vi "Minhee Analysis.vi"(5 "Data type":T4 items=["AXON", "HEKA", "TEXT"], 7 "Path of File":path=path "C:/Users/KimYG/Desktop/test4.abf") -> ()   [LabVIEW 2017] (continued)
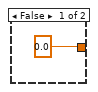
[diagram p4: hidden frame]
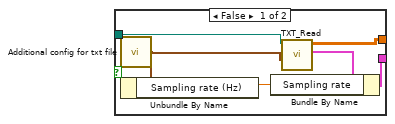
[diagram p5: hidden frame]
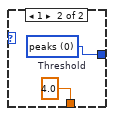
[diagram p6: hidden frame]
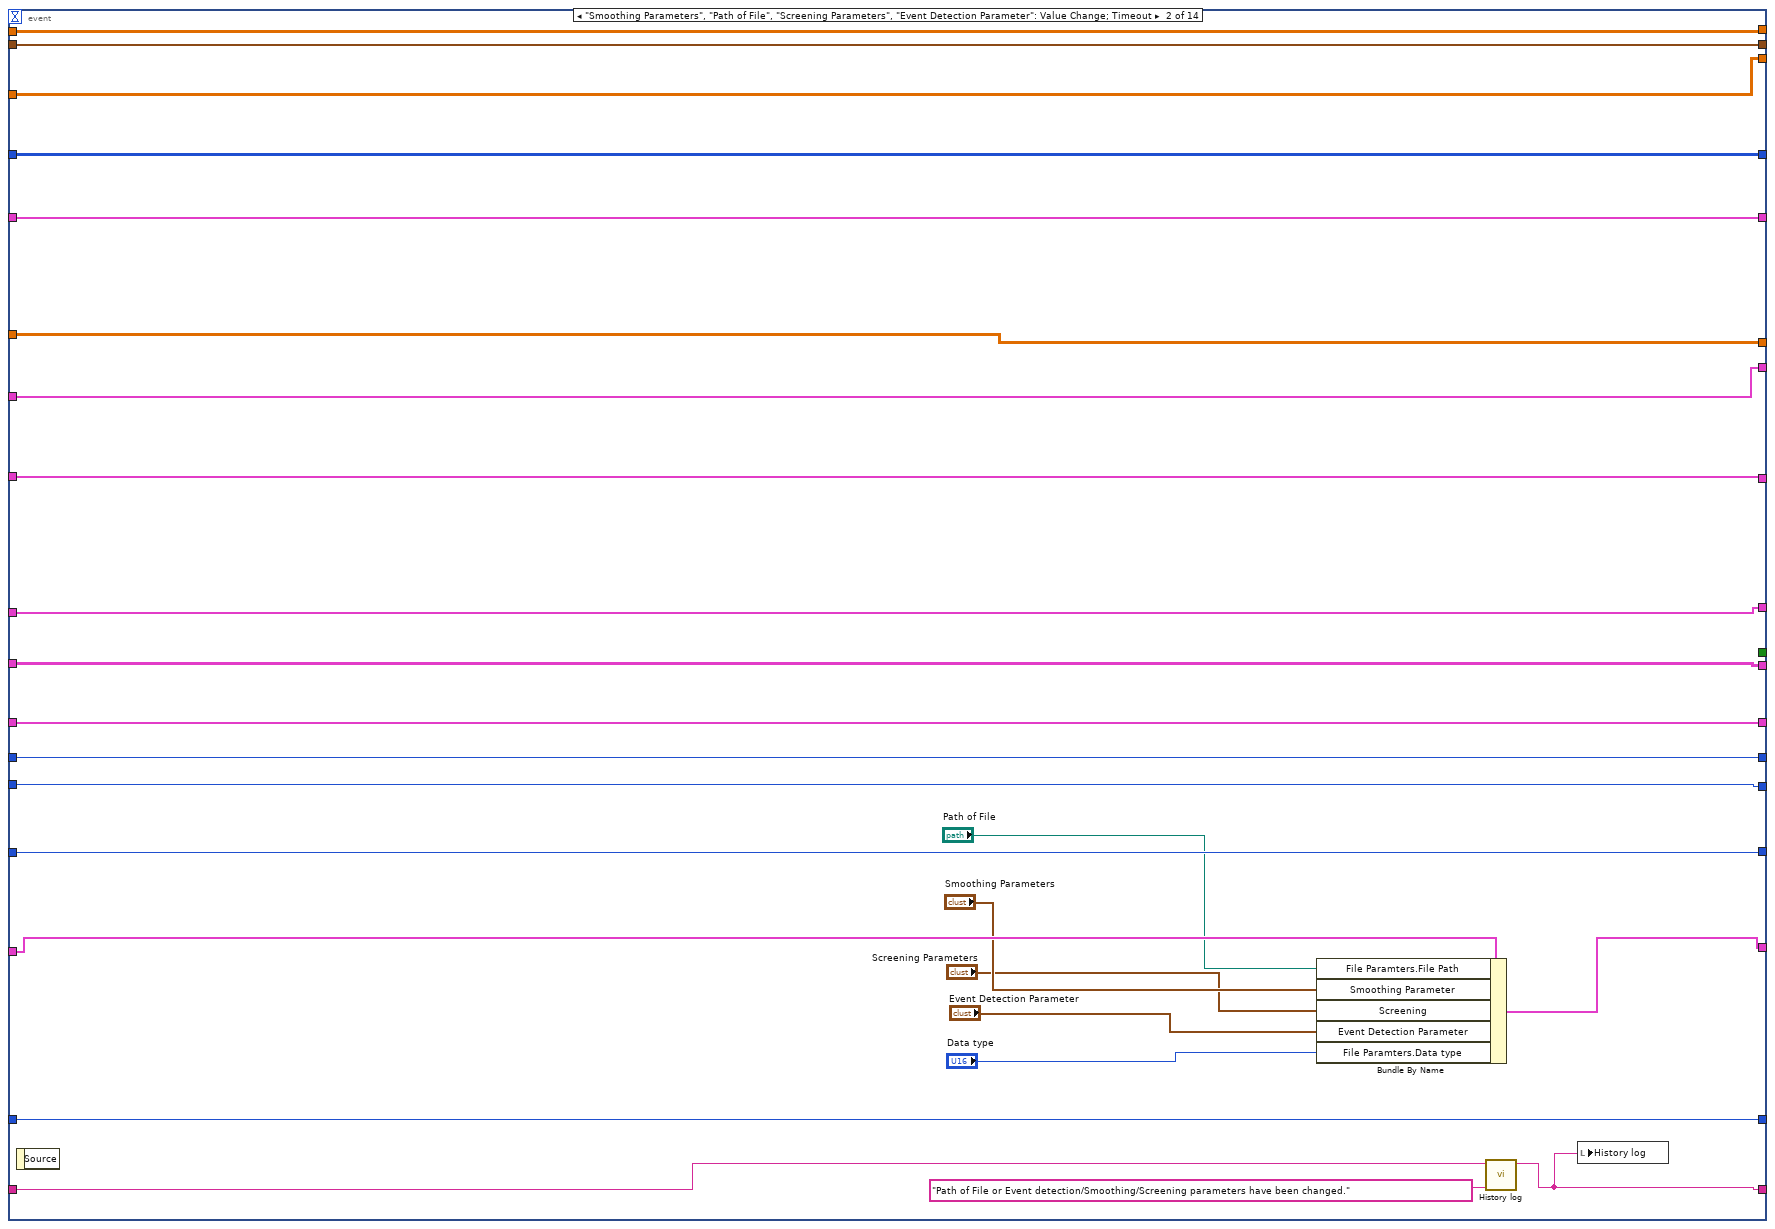
[diagram p7: hidden frame]
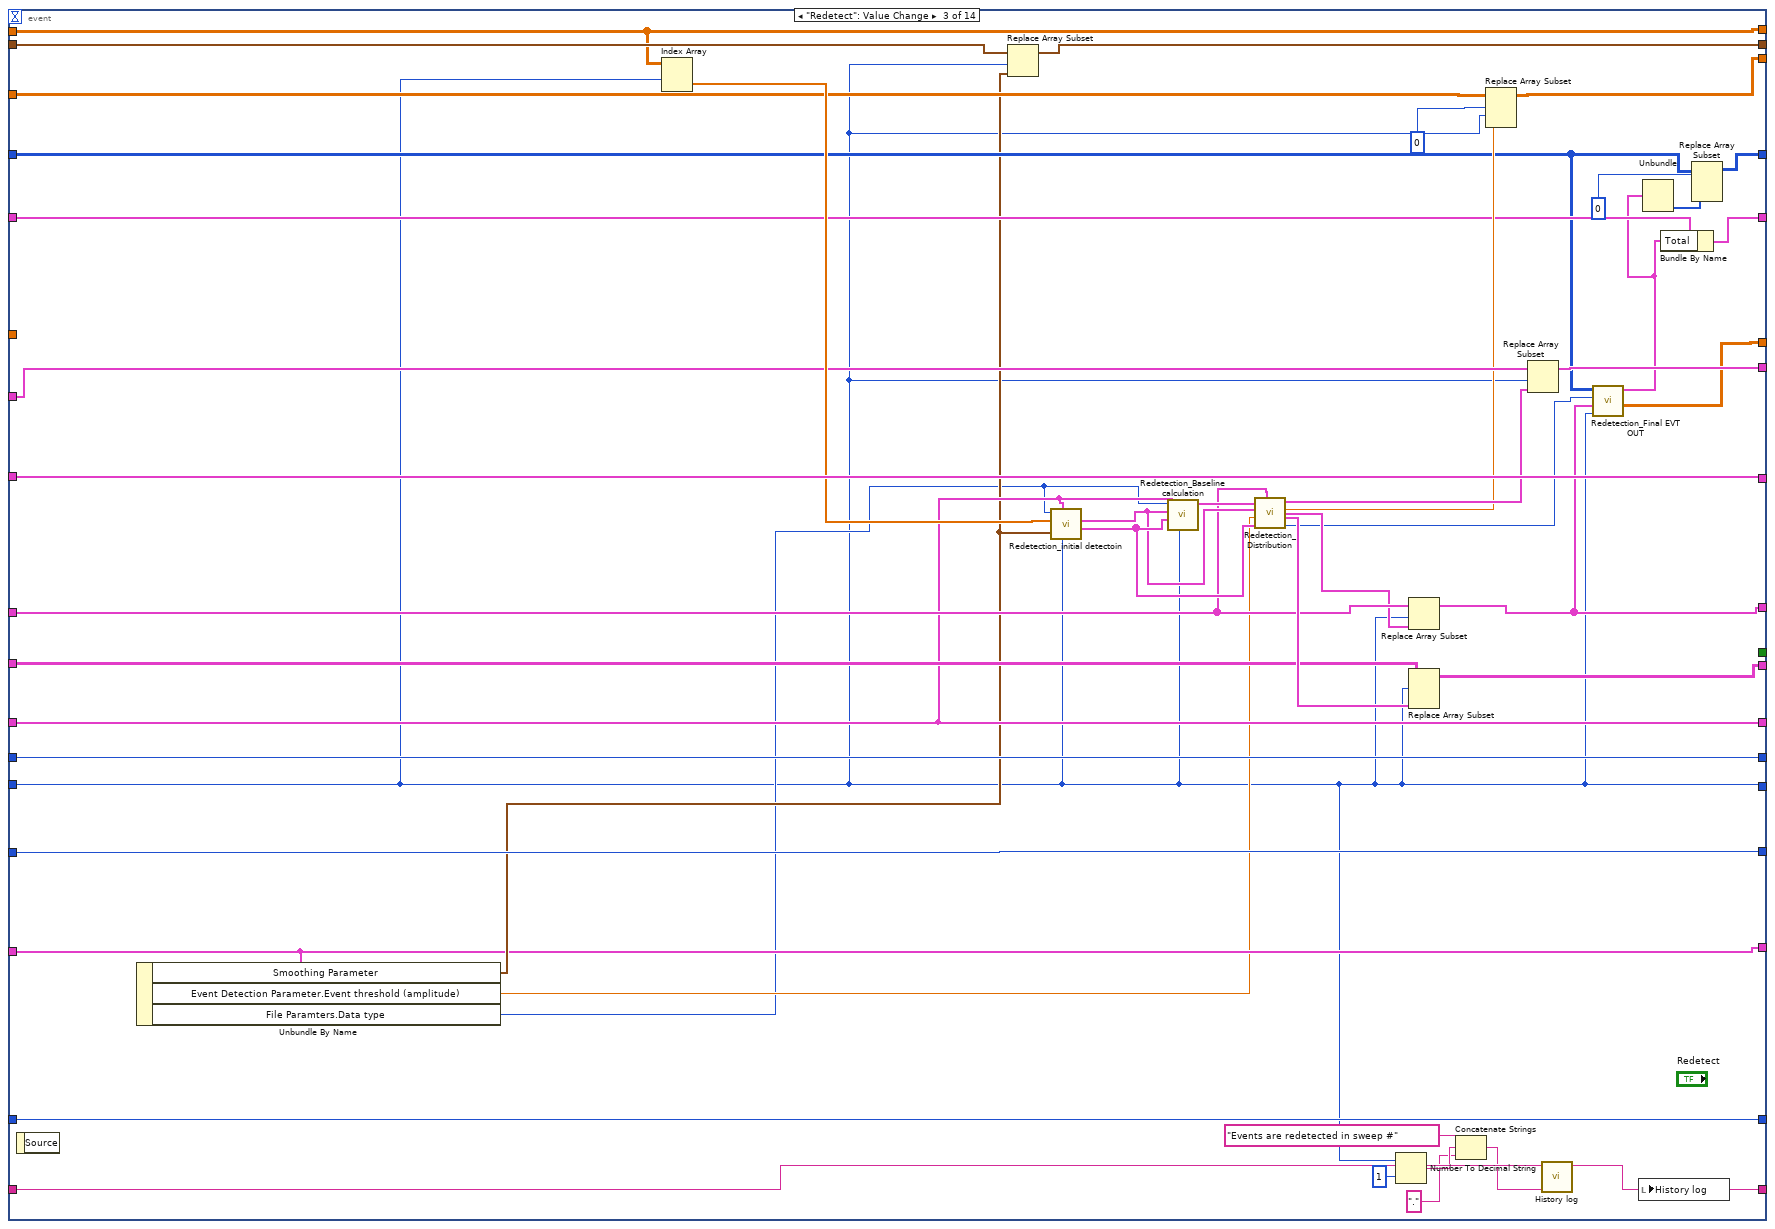
[diagram p8: hidden frame]
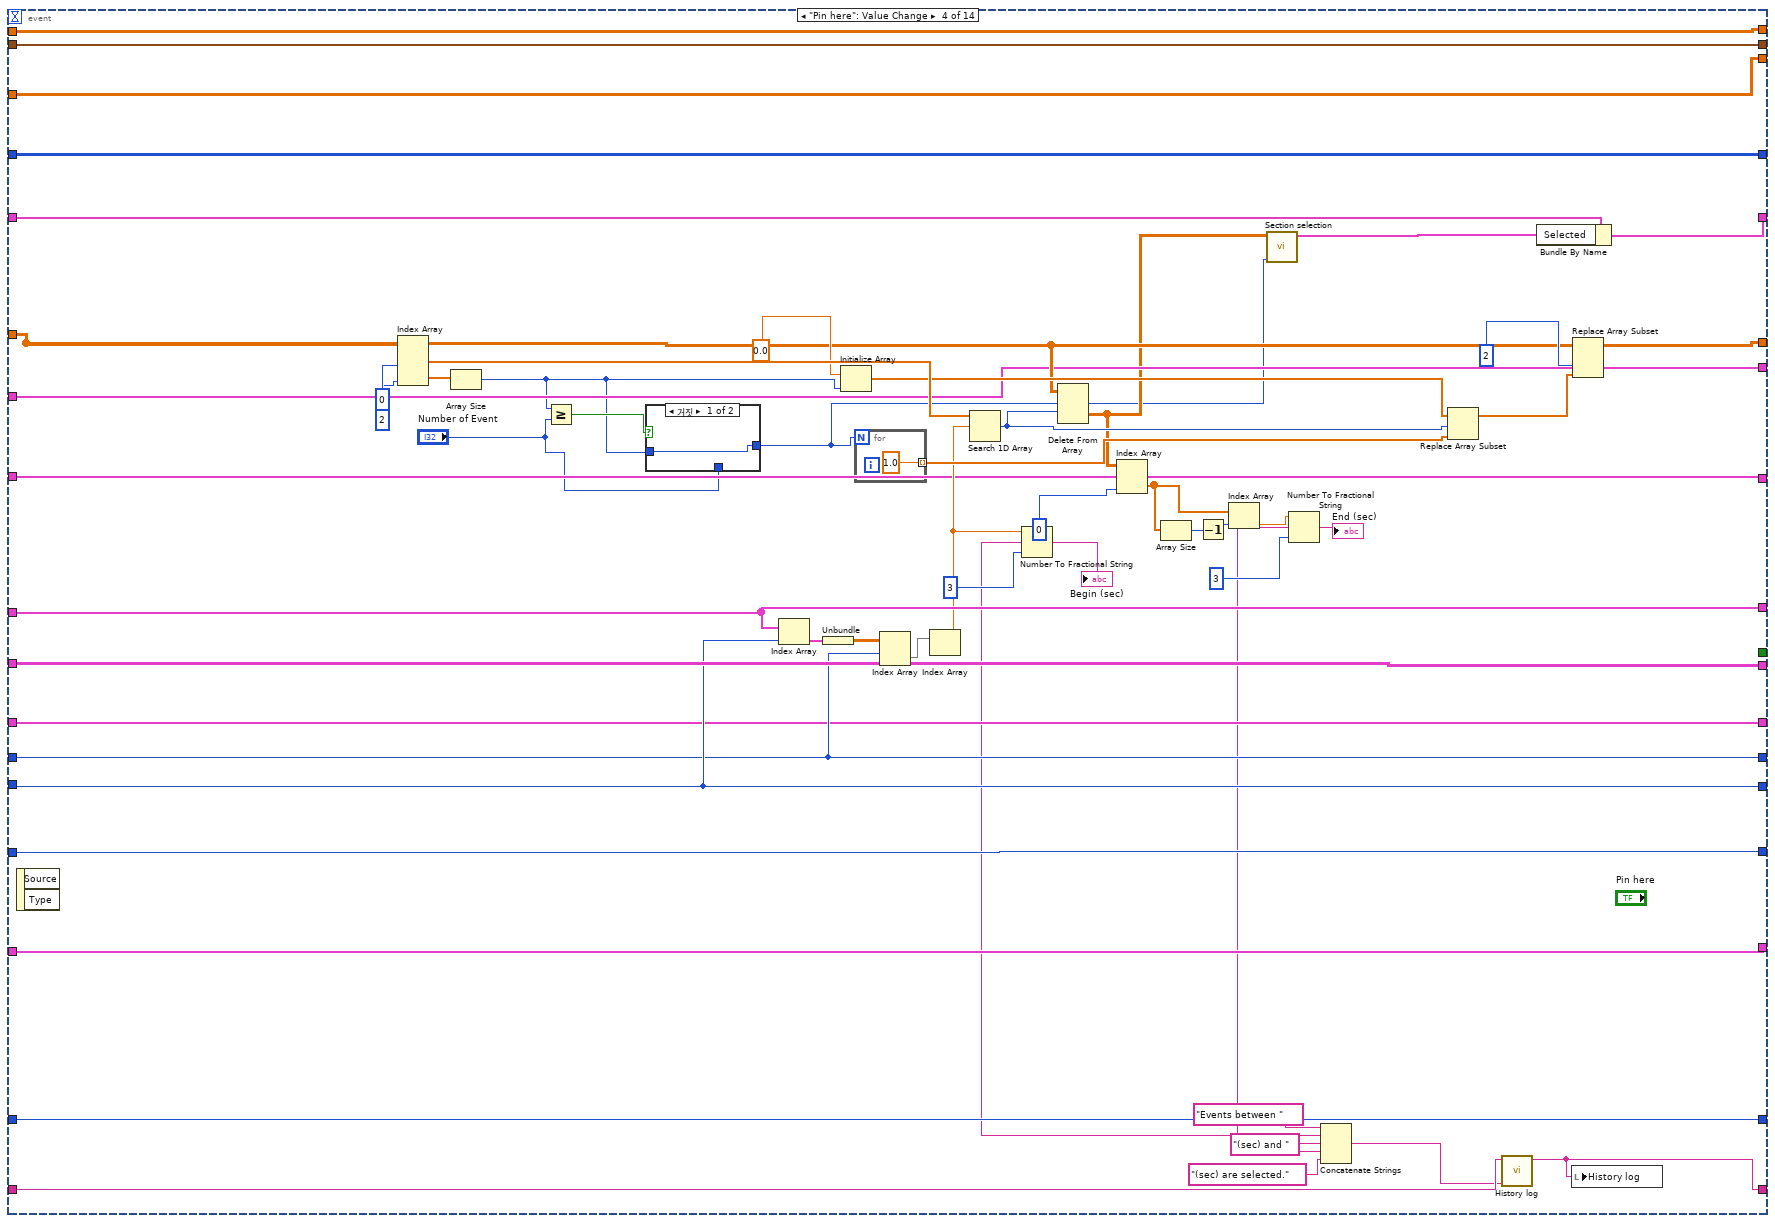
[diagram p9: hidden frame]
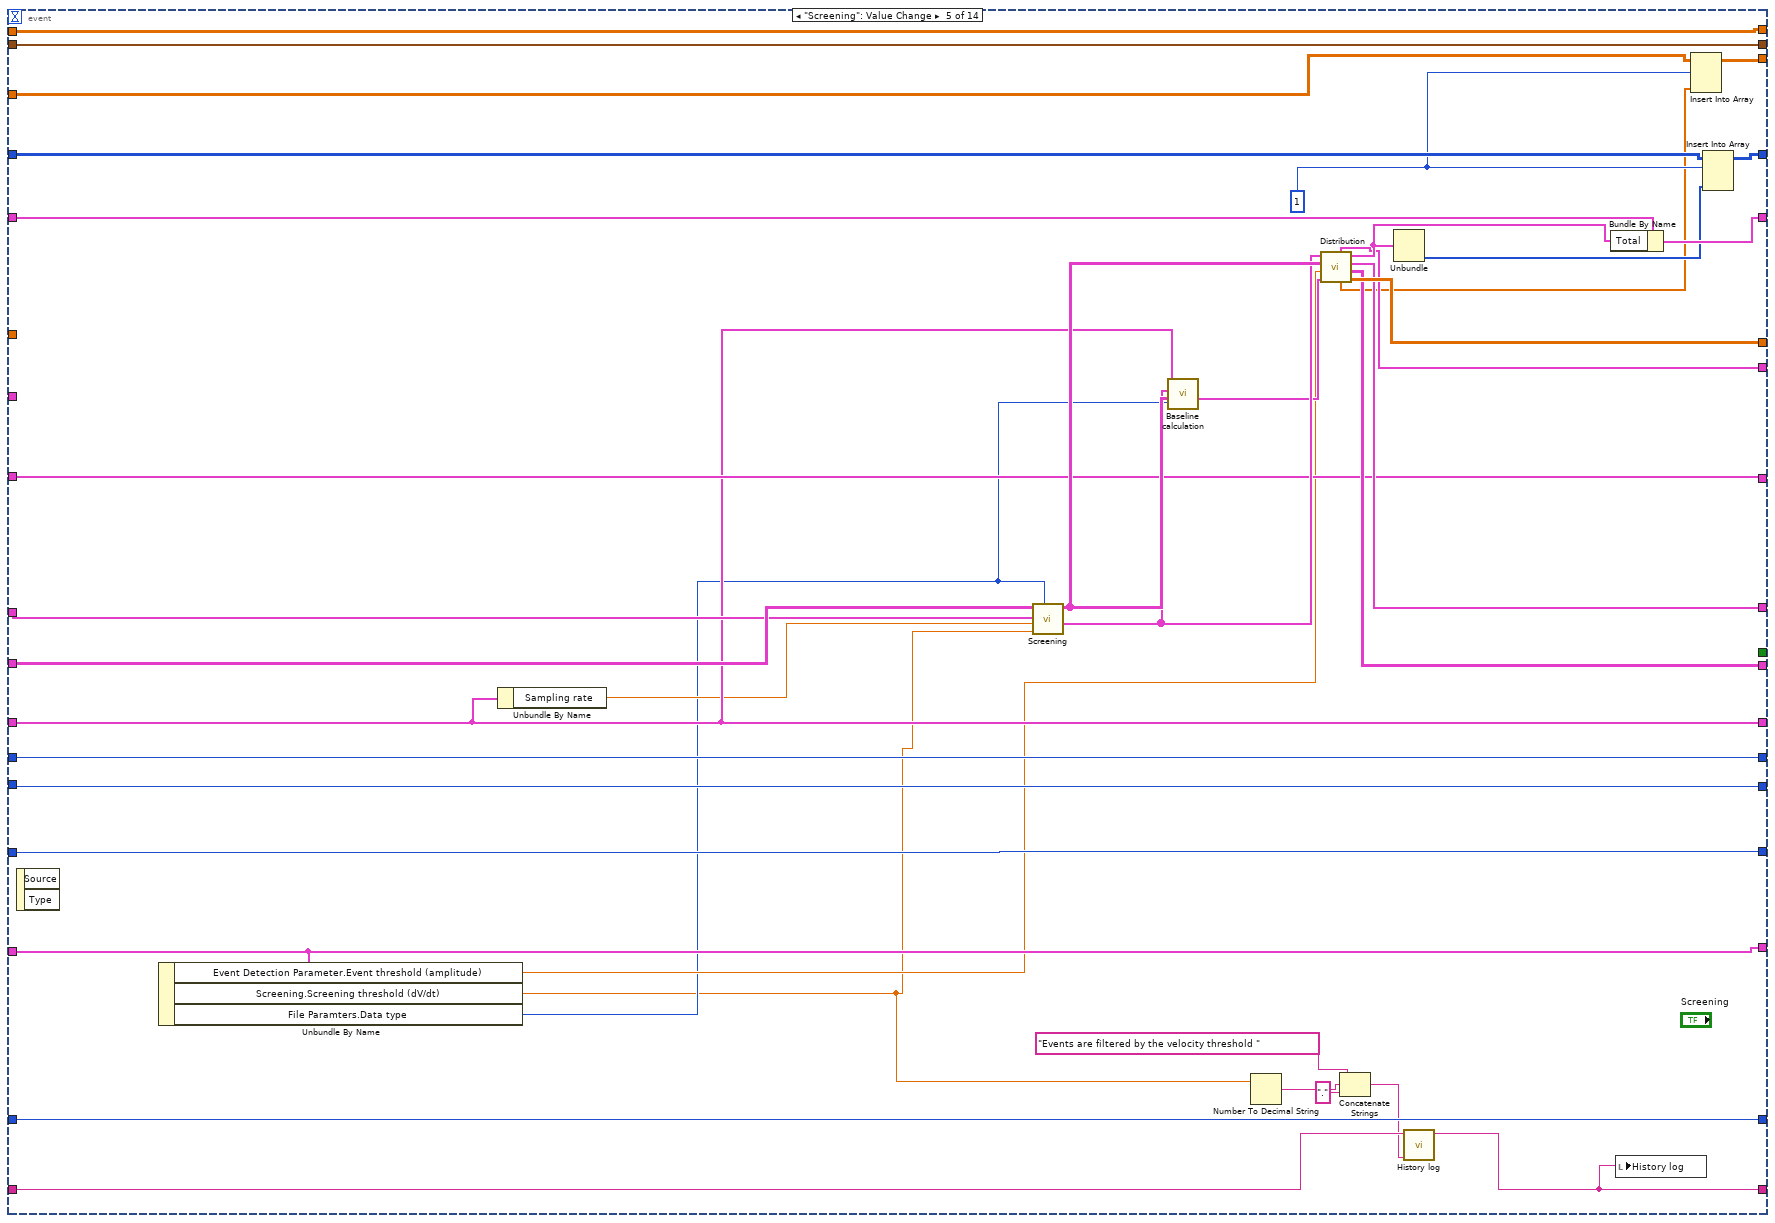
[diagram p11: hidden frame]
            n155 = Number To Decimal String(number=w476) -> (decimal integer string=w474:string)  [unwired: 1 in]
            n156 = call "Distribution.vi"("Detected Event IN"=w497, "Sweep trace (2D) In"=w491, "Threshold"=w479, "Baseline info IN"=w492) -> ("Baseline info new OUT"=w488:cluster{dbl[][]}[], "Distribution (output)"=w495:T15, "Detected Event (1D) OUT"=w489:cluster{dbl[][]}[], "Sweep trace (2D) Out"=w490:cluster{"Ramp Pattern":dbl[], "X":dbl[]}[][], "Event final OUT"=w496:dbl[][])  [unwired: 1 out]
            n157 = Concatenate Strings("Event is deleted. ", " (Event #", w474, " in Sweep #", w471, ")" ("문자열")) -> (w469:string)
            n158 = call "History log.vi"("Message"=w469, "String IN"=w477) -> ("String OUT"=w468:string)  [unwired: 5 in]
            n159 = local write "History log"(w468) -> ()
            n160 = Bundle By Name(cluster=w494, "Total"=w495) -> (w493:T7)
          }
          event "Clipboard": Value Change {
            n161 = event-data() -> ()  [unwired: 1 in, 2 out]
            n162 = Unbundle By Name(w505) -> ("File Paramters.Data type"=w504:T4)
            n163 = case shown="1" w504 {
              tunnel: w513 -> [w526 w533]
              tunnel: [w526 w532] -> w514
              frame 0, Default {
              }
              frame 1 {
                n164 = Index Array(array=w533, index (col)=0 ("비활성화된 인덱스 (열)")) -> (element=w530:dbl[])  [unwired: 1 in]
                n165 = Divide(x=w530, y=2.0 ("x")) -> (x/y=w528:dbl[])
                n166 = Replace Array Subset(array=w533, new element=w528, index (col)=0 ("비활성화된 인덱스 (열)")) -> (w532:dbl[][])  [unwired: 1 in]
              }
            }
            n167 = Number To Exponential String(number=w514) -> (E-format string=w516:string[][])  [unwired: 3 in]
            n168 = call <userlib>:"Clipboard transformation.vi"("Input (structured)"=w516) -> ("Output (flattened)"=w517:string)  [unwired: 1 in, 1 out]
            n169 = Open Application Reference() -> (0:w519:errorcluster)  [unwired: 4 in, 1 out]
            n170 = invoke class="App" method="Clipboard.Write"(error in=w519, "Param 0"=w517) -> (reference out=w518:refnum<vi>)  [unwired: 2 in, 3 out]
            n171 = call "History log.vi"("Message"="Events are exported to clipboard.", "String IN"=w503) -> ("String OUT"=w501:string)  [unwired: 5 in]
            n172 = Close Reference(reference=w518) -> ()  [unwired: 1 in, 1 out]
            n173 = local write "History log"(w501) -> ()
          }
          event "Event #": Value Change {
            n174 = event-data() -> ()  [unwired: 1 in, 1 out]
          }
          event "Trace to display", "Derivative": Value Change {
            n175 = event-data() -> ()  [unwired: 1 in, 1 out]
          }
          event "File Explorer": Value Change {
            n176 = event-data() -> ()  [unwired: 1 in, 1 out]
            n177 = Unbundle By Name(w570) -> ("File Paramters.File Path"=w569:path)
            n178 = call <vilib>:"Show in File System.vi"("file or directory path"=w569) -> ()  [unwired: 10 in, 1 out]
          }
          event "Raw trace": Value Change {
            w605 = TRUE ("눈금 숨기기")
            n179 = event-data() -> ()  [unwired: 1 in, 2 out]
            n180 = Index Array(array=w614, index (row)=w613) -> (element=w612:cluster{"Ramp Pattern":dbl[], "X":dbl[]}[])  [unwired: 1 in]
            n181 = Index Array(array=w612, index=1 ("인덱스")) -> (element=w610:cluster{"Ramp Pattern":dbl[], "X":dbl[]})
            n182 = Unbundle(w610) -> ("Ramp Pattern"=w609:dbl[], "X"=w608:dbl[])
            n183 = Build Array(w609, w608) -> (w607:dbl[][])
            n184 = call-poly <vilib>:"Write Delimited Spreadsheet.vi"("2D data"=w607, "transpose? (no:F)"=TRUE ("transpose? (F)")) -> ("new file path (Not A Path if cancelled)"=w602:path, "error out"=w598:errorcluster)  [unwired: 12 in]
            n185 = Strip Path(path=w602) -> (stripped path=w601:path)  [unwired: 1 out]
            n186 = Build Path(base path=w601, name or relative path="Raw trace.bmp" ("이름 또는 상대 경로")) -> (appended path=w599:path)
            n187 = invoke on="Whole trace" class="XYGraph (엄격한)" method="Export Image"(error in=w598, "FileType"=enum32{"BMP", "EPS", "EMF", "PICT"}."BMP" ("파일 타입"), "Target"=enum32{"File", "Clipboard"}."File" ("타겟"), "Path"=w599, "HideGrid"=w605, "Overwrite"=w605) -> ()  [unwired: 2 in, 8 out]
          }
          event "Save": Value Change {
            n188 = event-data() -> ()  [unwired: 1 in, 2 out]
            n189 = Unbundle By Name(w627) -> ("File Paramters.File Path"=w626:path, "File Paramters.Data type"=w625:T4)
            n190 = Strip Path(path=w626) -> (stripped path=w644:path, name=w640:string)
            n191 = case shown="0, 기본" w625 {
              tunnel: w642 -> [w654 w661]
              tunnel: [w654 w660] -> w641
              frame 0, Default {
              }
              frame 1 {
                n192 = Index Array(array=w661, index (col)=0 ("비활성화된 인덱스 (열)")) -> (element=w658:dbl[])  [unwired: 1 in]
                n193 = Divide(x=w658, y=2.0 ("x")) -> (x/y=w656:dbl[])
                n194 = Replace Array Subset(array=w661, new element=w656, index (col)=0 ("비활성화된 인덱스 (열)")) -> (w660:dbl[][])  [unwired: 1 in]
              }
            }
            n195 = To Lower Case(string=w640) -> (all lower case string=w639:string)
            n196 = Match Pattern(string=w639, regular expression="abf" ("정규식")) -> (before substring=w647:string)  [unwired: 1 in, 3 out]
            n197 = Concatenate Strings(w647, "txt" ("문자열")) -> (w645:string)
            n198 = Build Path(base path=w644, name or relative path=w645) -> (appended path=w643:path)
            n199 = call-poly <vilib>:"Write Delimited Spreadsheet.vi"("file path (dialog if empty)"=w643, "format (%.3f)"="%.5f", "2D data"=w641, "transpose? (no:F)"=FALSE ("transpose? (F)")) -> ("new file path (Not A Path if cancelled)"=w623:path)  [unwired: 10 in, 1 out]
            n200 = Path To String(path=w623) -> (string=w621:string)
            n201 = Concatenate Strings("Event file is saved. (file path: ", w621, ")") -> (w619:string)
            n202 = call "History log.vi"("Message"=w619, "String IN"=w624) -> ("String OUT"=w618:string)  [unwired: 5 in]
            n203 = local write "History log"(w618) -> ()
          }
          event Panel Close? {
            n204 = event-data() -> ()  [unwired: 1 in, 4 out]
            n205 = Two Button Dialog(message="Are you sure you want to quit?" ("메시지"), 1:"Cancel" ("거짓 버튼 이름(\"취소\")"), 2:"Yes" ("참 버튼 이름(\"확인\")")) -> (T button?=w683:bool)
            n206 = case shown="참" w683 {
              tunnel: [FALSE TRUE] -> w701
              tunnel: w699 -> [w720 _]
              tunnel: w698 -> [w719 _]
              tunnel: w697 -> [w718 _]
              tunnel: w696 -> [w717 _]
              tunnel: w695 -> [w715 _]
              tunnel: w694 -> [w714 w729]
              tunnel: w693 -> [w713 w728]
              tunnel: [w720 _] -> w692
              tunnel: [w719 _] -> w691
              tunnel: [w718 _] -> w690
              tunnel: [w717 _] -> w689
              tunnel: w688 -> [w716 w724]
              tunnel: [w716 w724] -> w687
              tunnel: [w715 _] -> w686
              tunnel: [w714 w729] -> w685
              tunnel: [w713 w728] -> w684
              tunnel: w682 -> [w711 _]
              tunnel: [w711 _] -> w681
              tunnel: w680 -> [w710 _]
              tunnel: [w710 _] -> w679
              tunnel: w678 -> [w709 _]
              tunnel: [w709 _] -> w677
              tunnel: w676 -> [w708 _]
              tunnel: [w708 u16 0 ("Trace to display")] -> w675
              tunnel: w674 -> [w707 _]
              tunnel: [w707 _] -> w673
              tunnel: w672 -> [w706 _]
              tunnel: [w706 _] -> w671
              tunnel: w670 -> [w705 _]
              tunnel: [w705 _] -> w669
              tunnel: w666 -> [w704 _]
              tunnel: [w704 _] -> w665
              tunnel: w664 -> [w703 w722]
              tunnel: [w703 w722] -> w663
              tunnel: [TRUE TRUE] -> w662
              frame False {
              }
              frame True {
                w725 = ""
                w726 = dbl[] [] ("CV")
                n207 = property on="Begin (sec)" class="Str"("Value"=w725) -> ()  [unwired: 2 in, 2 out]
                n208 = property on="End (sec)" class="Str"("Value"=w725) -> ()  [unwired: 2 in, 2 out]
                n209 = property on="CV" class="WFGraph (엄격한)"("Value"=w726) -> ()  [unwired: 2 in, 2 out]
                n210 = property on="Holding Current" class="WFGraph (엄격한)"("Value"=w726) -> ()  [unwired: 2 in, 2 out]
              }
            }
            n211 = event-data("Discard?"=w662) -> ()  [unwired: 1 in, 1 out]
          }
        }
        "Number of event" <- w89
        "Averaged Amplitude" <- w62
        n212 = Unbundle By Name(w103) -> ("Total.Distribution of IEI"=→"Distribution of IEI":T5, "Total.Distribution of amplitude"=→"Distribution of amplitude":T5, "Total.Total"=w100:T19, "Selected.Distribution of IEI"=→"Distribution of IEI 2":T5, "Selected.Distribution of amplitude"=→"Distribution of amplitude 2":T5, "Selected.Selected"=w94:T20)
        n213 = Unbundle By Name(w34) -> ("Screening.Screening threshold (dV/dt)"=w33:dbl, "File Paramters.Data type"=w32:T4)
        n214 = Unbundle By Name(w87) -> ("Sampling rate"=w86:dbl)
        n215 = Index Array(array=w137, index (row)=w37) -> (element=w73:cluster{"Ramp Pattern":dbl[], "X":dbl[]}[])  [unwired: 1 in]
        n216 = Index Array(array=w73, index=2 ("인덱스")) -> (element=w112:cluster{"Ramp Pattern":dbl[], "X":dbl[]})
        n217 = local read "Sweep duration"() -> (w84:dbl)
        n218 = Unbundle By Name(w112) -> ("X"=w66:dbl[])
        n219 = Index Array(array=w73, index #1=0 ("인덱스"), index #2=2 ("인덱스"), index #3=1 ("인덱스")) -> (element #1=w70:cluster{"Ramp Pattern":dbl[], "X":dbl[]}, element #2=w68:cluster{"Ramp Pattern":dbl[], "X":dbl[]}, element #3=w58:cluster{"Ramp Pattern":dbl[], "X":dbl[]})
        n220 = Index Array(array=w71, index=w37) -> (element=w60:cluster{dbl[], dbl[]})
        n221 = Reciprocal(x=w86) -> (1/x=w85:dbl)
        n222 = case shown="0, 기본" w56 {
          tunnel: w60 -> [w147 _]
          tunnel: [w147 w148] -> w59
          tunnel: w58 -> [_ w148]
          frame 0, Default {
          }
          frame 1 {
          }
        }
        n223 = Array Max & Min(array=w66) -> (max value=w64:dbl, min value=w65:dbl)  [unwired: 2 out]
        n224 = Build Array(w70, w59, w68) -> (→"Whole trace":cluster{"Ramp Pattern":dbl[], "X":dbl[]}[])
        n225 = Multiply(x=w37, y=w84) -> ()  [unwired: 1 out]
        n226 = Add(x=-80.0, y=w65) -> (x+y=w106:dbl)
        n227 = Add(x=w64, y=40.0 ("x")) -> (x+y=w105:dbl)
        n228 = Index Array(array=w133, index=w37) -> (element=w140:cluster{dbl[][]})
        n229 = Unbundle(w94) -> ("EVT #"=→"Event #":string, "Amplitude"=→"Amplitude\n     (pA)":string, "IEI"=→"IEI (sec)":string, "Frequency"=→"Frequency":string)
        n230 = call "View.vi"("dt"=w85, "Data type"=w32, "Event #"=w120, "Sweep #"=w37, "Baseline info new OUT"=w76, "Sweep trace (2D) In"=w137, "Detected Event (1D) In"=w133) -> ("event"=→"Event":cluster{dbl[], dbl[]}[], "출력 클러스터"=w136:T21)  [unwired: 1 in, 1 out]
        n231 = Unbundle(w100) -> ("EVT #"=→"Event #":string, "Amplitude"=→"Amplitude\n     (pA)":string, "IEI"=→"IEI (sec)":string)
        n232 = Unbundle(w140) -> (w39:dbl[][])
        n233 = Index Array(array=w39, index (col) #1=0 ("비활성화된 인덱스 (열)"), index (col) #2=3 ("인덱스 (열)")) -> (element #1=w42:dbl[], element #2=w41:dbl[])  [unwired: 2 in]
        n234 = Unbundle(w136) -> ("X (time)"=w132:dbl[], "1st derivative"=w49:dbl[], "2nd derivative"=w47:dbl[])  [unwired: 1 out]
        n235 = property on="History log" class="Str"("Text.Scroll Position"=u32 4294967295 ("텍스트.스크롤 위치")) -> ()  [unwired: 2 in, 2 out]
        n236 = Build Array(w42, w41) -> (w40:dbl[][])
        n237 = Transpose 2D Array(2D array=w40) -> (transposed array=w38:dbl[][])
        n238 = Number To Fractional String(number=w38, precision (6)=i16 3 ("폭(-)")) -> (F-format string=w123:string[][])  [unwired: 2 in]
        "Event table" <- w123
        n239 = case shown="1" w50 {
          tunnel: w49 -> [w145 _]
          tunnel: [w145 w146] -> w48
          tunnel: w47 -> [_ w146]
          frame 0, Default {
          }
          frame 1 {
          }
        }
        n240 = for {
          tunnel: w49 -> [_] mode=indexing
          tunnel: [w149] -> w131 mode=indexing
          tunnel: w33 -> [w149]
        }
        n241 = Array Size(array=w123) -> (size(s)=w135:i32[])
        n242 = Bundle("X (time)"=w132, "2nd derivative"=w48) -> (w129:T22)  [unwired: 1 in]
        n243 = Index Array(array=w135, index=0 ("인덱스 (행)")) -> (element=w127:i32)
        n244 = Bundle("X (time)"=w132, w131) -> (w130:cluster{"X (time)":dbl[], dbl[]})  [unwired: 1 in]
        n245 = Decrement(x=w127) -> (x-1=w126:i32)
        n246 = Index Array(array=w39, index (row)=w120) -> (element=w122:dbl[])  [unwired: 1 in]
        n247 = property on="Event #" class="DigNum (엄격한)"("Maximum"=w126, "Minimum"=0.0 ("데이터 입력 제한:최소")) -> ()  [unwired: 2 in, 2 out]
        n248 = Build Array(w129, w130) -> (→"Derivative of the event":T23)
        n249 = Index Array(array=w122) -> (element #1=w78:dbl, element #2=w79:dbl)  [unwired: 2 in]
        n250 = Round Toward +Infinity(x=w106) -> (ceil(x): smallest int >= x=w82:dbl)
        n251 = property on="Averaged Amplitude" class="WFGraph (엄격한)"("Active Cursor"=u32 0 ("활성 커서"), "Cursor.Cursor X"=w37) -> ()  [unwired: 2 in, 2 out]
        n252 = property on="Number of event" class="WFGraph (엄격한)"("Active Cursor"=u32 0 ("활성 커서"), "Cursor.Cursor X"=w37) -> ()  [unwired: 2 in, 2 out]
        n253 = Round Toward +Infinity(x=w105) -> (ceil(x): smallest int >= x=w81:dbl)
        n254 = property on="Holding Current" class="WFGraph (엄격한)"("Active Cursor"=u32 0 ("활성 커서"), "Cursor.Cursor X"=w37) -> ()  [unwired: 2 in, 2 out]
        n255 = Bundle(cluster=w116, "Row"=w120, "Column"=u32 0 ("활성 커서")) -> (w75:T12)
        n256 = Bundle(cluster=w116, "Row"=u32 1 ("활성 커서"), "Column"=u32 2 ("활성 커서")) -> (w119:T12)
        n257 = property on="Whole trace" class="XYGraph (엄격한)"("Active Cursor"=u32 0 ("활성 커서"), "Cursor.Cursor X"=w78, "YScale.Minimum"=w82, "YScale.Maximum"=w81) -> ()  [unwired: 2 in, 2 out]
        n258 = property on="Derivative of the event" class="XYGraph (엄격한)" props=["Active Cursor", "Cursor", "Cursor X", "Cursor", "Cursor Y", "Width"]("Active Cursor"=u32 0 ("활성 커서"), "Cursor.Cursor X"=w78, "Cursor.Cursor Y"=w79) -> ()  [unwired: 2 in, 3 out]
        n259 = property on="Event table" class="Tbl (엄격한)"("Selection Start"=w75, "Selection Size"=w119, "Selection Color"=u32 16722664) -> ()  [unwired: 2 in, 2 out]
        n260 = property on="Event" class="XYGraph (엄격한)"("Active Cursor"=u32 0 ("활성 커서"), "Cursor.Cursor X"=w78, "Cursor.Cursor Y"=w79) -> ()  [unwired: 2 in, 2 out]
      }
    }
    frame #2 {
      n261 = local read "StateFileRefnum"() -> (w730:T3)
      n262 = Current VI's Path ("Current VI's Path...")() -> (path=w734:path)
      n263 = Open VI Reference(vi path=w734) -> (vi reference=w733:refnum<vi>)  [unwired: 5 in, 1 out]
      n264 = call <userlib>:"SaveVIState.vi"("StateFileRefnum"=w730, "key"="StateKey", "VI Refnum"=w733) -> ()
      n265 = property class="App"() -> ("App.Kind"=w731:T24)  [unwired: 2 in, 2 out]
      n266 = case shown="\"Run Time System\"" w731 {
        frame "invalid app kind", Default {
        }
        frame "Development System" {
        }
        frame "Run Time System" {
          n267 = Quit LabVIEW() -> ()  [unwired: 1 in]
        }
      }
    }
  }
  n268 = call <vilib>:"Close Config Data.vi"("write file if changed (T)"=TRUE ("write configuration file? (F)"), "refnum"=w1) -> ()  [unwired: 8 in, 2 out]